vi "UHR-Fleezers Control (host) - 12.7.vi"() -> ()   [LabVIEW 2012] (continued)
  T21 = enum16{"empty", "write", "read oldest (queue)", "read newest (stack)", "read all"}
  T22 = cluster{"New Image":T2, "New Image":T2, "New Image":T2, "New Image":T2, "New Image":T2}
  T23 = typedef "XDNodeRunTimeDep.lvlib/timing_clust.ctl" = cluster{"Expected End [f-1]":u64, "Actual End [f-1]":u64, "Finished Late? [f-1]":bool, "Expected End [i-1]":u64, "Actual End [i-1]":u64, "Finished Late? [i-1]":bool, "Expected Start [i]":u64, "Actual Start [i]":u64, "Expected Start [f]":u64, "Actual Start [f]":u64, "Source Name":string, "Structure Name":string, "Period":i64, "Deadline":i64, "Offset":i64, "Start":i64, "Priority":i32, "Timeout":i32, "Mode":T24, "Wakeup Reason":T25, "Error":errorcluster, "Source Type":string, "Secondary Source Type":string, "Global End Time":u64, "Global Start Time":u64, "Frame Duration":u64, "Iteration Duration":u64, "Assigned CPU":i32, "I/O Scan Engine Mode":u32}
  T24 = typedef "XDNodeRunTimeDep.lvlib/nitl_modes.ctl" = enum32{"No Change", "Process missed periods, maintain original phase", "Discard missed periods, maintain original phase", "Process missed periods, ignore original phase", "Discard missed periods, ignore original phase"}
  T25 = typedef "XDNodeRunTimeDep.lvlib/wakeup.ctl" = enum32{"Normal", "Aborted", "Asynchronous wakeup", "Timing source error", "Timed loop error", "Timeout"}
  T26 = enum32{"Status", "Sample Stage", "Syringe Pump", "Trap Control (RF)", "APD Counting", "Fluorescence Laser Control", "Trap AI", "Video", "FPGA"}
  T27 = enum32{"Status", "Sample Stage", "Syringe Pump", "Trap Control (RF)", "APD Counting", "Fluorescence Laser Control", "Trap AI", "Video", "FPGA", "Misc. Configuration"}
  T28 = enum16{"big-endian, network order", "native, host order", "little-endian"}
  T29 = enum16{"open", "replace", "create", "open or create", "replace or create", "replace or create with confirmation"}
  T30 = cluster{"Scan Range AOD (nm) 2":dbl, "Step Size AOD (nm) 2":dbl, "Scan Speed AOD (nm/s) 2":dbl, "Number of scans (AOD) 2":u16, "Label":string}
  T31 = cluster{"[0]":dbl, "[1]":dbl, "[2]":dbl, "[3]":dbl, "[4]":dbl, "[5]":dbl}
  T32 = cluster{"Diameter (mm)":dbl, "Units":dbl, "Volume":dbl, "Rate":dbl}
  T33 = cluster{"Left":i32, "Top":i32, "Width":u32, "Height":u32}
  T34 = cluster{cluster{"Left":i32, "Top":i32, "Width":u32, "Height":u32}}[]
  T35 = enum32{"Normal Display", "Dual Display (APD)", "FFT", "High Res Display"}
  T36 = cluster{"Origin Pixel":cluster{"X":sgl, "Y":sgl}, "Angle Relative to Horizontal (deg)":sgl, "Axis Reference":u32}
  T37 = typedef "Simple Grid Descriptor" = cluster{"X Step":sgl, "Y Step":sgl, "Unit":T38}
  T38 = typedef "Image Unit" = enum32{"Undefined", "Angström", "Micrometer", "Millimeter", "Centimeter", "Meter", "Kilometer", "Microinch", "Inch", "Feet", "Nautical miles", "Standard miles", "Steps"}
  T39 = cluster{"averaging mode":u16, "weighting mode":u16, "number of averages":u32}
  T40 = cluster{"dB On (F)":bool, "unwrap phase (F)":bool, "convert to degree (F)":bool}
  T41 = cluster{string, string, string, string, string, string, string, string}
  T42 = cluster{string, string, string, string, string, string, string, string, string, string, string, string}
  T43 = cluster{string, string, string, string, string, string, string, string, string, string, string, string, string}
  T44 = cluster{string, string, string, string, string, string, string, string, string, string, string, string, string, string}
  T45 = cluster{"BD 1 Frequency 1 (MHz)":dbl, "BD 1 Frequency 2 (MHz)":dbl}
  T46 = cluster{"f0":dbl, "df":dbl, "magnitude":dbl[]}[][]
  T47 = cluster{"Comment (data description)":string, "Channel 1 Buffer":string, "Channel 2 Buffer":string, "Channel 3 Buffer":string, "Title":string, "DNA Construct":string, "Bead diameter":dbl, "Name":string}
  T48 = enum32{"setting", "request", "request control", "info", "statistics", "system settings", "I/O sub system", "HRT control", "camera descriptions", "device specific data", "event sub system settings", "event sub system results", "image memory manager"}
  T49 = typedef "AviRefnum.ctl" = refnum<k1>
  T50 = typedef "imagedata.ctl" = cluster{"image type":i32, "image depth":i32, "image":u8[], "mask":u8[], "colors":u32[], "Rectangle":cluster{"left":i16, "top":i16, "right":i16, "bottom":i16}}
diagram:
  w8 = u16 10 items=["1.0"=10, "1.5"=15, "2.0"=20] ("stop bits (10: 1 bit)")
  w75 = u16 20 items=["1.0"=10, "1.5"=15, "2.0"=20] ("stop bits (10: 1 bit)")
  w78 = u16 20 items=["1.0"=10, "1.5"=15, "2.0"=20] ("stop bits (10: 1 bit)")
  w104 = u16 20 items=["1.0"=10, "1.5"=15, "2.0"=20] ("stop bits (10: 1 bit)")
  w14 = T18 2 items=["Grayscale (U8)", "Grayscale (I16)", "Grayscale (SGL)", "Complex (CSG)", "RGB (U32)", "HSL (U32)", "RGB (U64)", "Grayscale (U16)"] ("Image Type")
  w234 = 10.0 ("y")
  w233 = 32767.0 ("y")
  w249 = 6.0  # clock mult.
  w250 = 49152000.0  # TCXO frequ.
  # "What are these?"
  # "I don't think you need to do this.\nEverytime you want to adjust phase you always set this anyway.\nSince we removed the separate +/- controls.\n\nHaven't added for added fl lasers.  Should remove this code."
  # "Bottom 1 Harvard"
  # "Top 3 Harvard"
  # "Center Harvard"
  # "Bottom 1 Harvard"
  # "Top 3 Harvard"
  # "Center Harvard"
  n1 = Build Array("DIO count 1 (ticks)", "DIO count 2 (ticks)", "DIO count 3 (ticks)") -> (w155:u16[])
  n2 = xnode "Open FPGA VI Reference"("resource name"=T19 "750kHzDAQ") -> ("FPGA VI Reference Out"=w258:T20, "error out"=w257:errorcluster)  [unwired: 1 in]
  n3 = local read "AO1"() -> (w228:dbl)
  n4 = local read "AO2"() -> (w227:dbl)
  n5 = local read "Scan Increment (MHz)"() -> (w245:dbl)
  n6 = local read "Continuous MCL Scanning"() -> (w215:bool)
  n7 = local read "Fast Scan Dir"() -> (w214:bool)
  n8 = xnode "Invoke Method"("FPGA VI Reference In"=w258, "error in"=w257) -> ("FPGA VI Reference Out"=w18:T20, "error out"=w174:errorcluster)
  n9 = local read "Number of scans (MCL)"() -> (w216:u64)
  n10 = Multiply(x=w228, y=w233) -> (x*y=w230:dbl)
  n11 = Multiply(x=w227, y=w233) -> (x*y=w232:dbl)
  n12 = Divide(x=w230, y=w234) -> (x/y=w229:dbl)
  n13 = Divide(x=w232, y=w234) -> (x/y=w231:dbl)
  n14 = To Word Integer(number=w229) -> (16bit integer=w226:i16)
  n15 = To Word Integer(number=w231) -> (16bit integer=w225:i16)
  n16 = Not(x=w214) -> (.not. x?=w209:bool)
  n17 = local read "Cycles/step (MCL)"() -> (w217:u64)
  n18 = Multiply(x=w245, y=1000.0) -> (x*y=w252:dbl)
  n19 = local read "Scan steps (MCL)"() -> (w218:u64)
  n20 = local read "Desired Scan Incr (V)"() -> (w220:dbl)
  n21 = Scale By Power Of 2(n=48, x=w252) -> (x*2^n=w253:dbl)
  n22 = Unbundle By Name(cluster{"output high":i16, "output low":i16} {"output high"=3000, "output low"=0} ("FB output range 1")) -> ("output high"=w56:i16, "output low"=w55:i16)
  n23 = Multiply(x=w250, y=w249) -> (x*y=w248:dbl)
  n24 = Divide(x=w253, y=w248) -> (x/y=w247:dbl)
  n25 = local read "Setpoints (V)"() -> (w264:cluster{"Set 1":dbl, "Set 2":dbl})
  n26 = To Quad Integer(1:w247) -> (0:w244:i64)
  n27 = Divide(x=40000000.0, y="AI Count (ticks)") -> (x/y=w205:dbl)
  n28 = Multiply(x=w220, y=32767.0) -> (x*y=w222:dbl)
  n29 = local read "Trap Intensity PID Gains"() -> (w259:T9)
  n30 = local write "Trap Pos FIFO Timeout"(u16 0 ("Trap Pos FIFO Timeout")) -> ()
  n31 = local read "Number Interlace Sets"() -> (w148:u8)
  n32 = Split 1D Array(array=w155, index=w148) -> (first subarray=w157:u16[])  [unwired: 1 out]
  n33 = Add Array Elements(numeric array=w157) -> (sum=w156:u16)
  n34 = local read "# Samples/channel"() -> (w237:u32)
  n35 = local read "Number of F/B Scans (AOD)"() -> (w238:u16)
  n36 = local read "Not-Interlacing Set"() -> (w147:enum32{"Set 1", "Set 2", "Set 3"})
  n37 = To Unsigned Byte Integer(number=w147) -> (unsigned 8bit integer=w153:u8)
  n38 = Index Array(array=w155, index=w153) -> (element=w154:u16)
  n39 = local read "Feedback On/Off"() -> (w267:cluster{"Set 1":bool, "Set 2":bool})
  n40 = local read "BD 2 Delay (Ticks)"() -> (w1:u8)
  n41 = local read "BD 1 Delay (ticks)"() -> (w2:u8)
  n42 = local read "Scan steps (AOD)"() -> (w243:u64)
  n43 = local read "All FB On/Off"() -> (w268:bool)
  n44 = local read "Cycles/step (AOD)"() -> (w242:u64)
  n45 = local write "AI rate (Hz)"(w205) -> ()
  n46 = Divide(x=w222, y=10.0) -> (x/y=w221:dbl)
  n47 = Multiply(x=w243, y=w242) -> (x*y=w241:u64)
  n48 = Unbundle By Name(w259) -> ("proportional gain (Kc)"=w60:i16, "integral gain (Kc*Ts/Ti)"=w59:i16, "derivative gain (Kc*Td/Ts)"=w58:i16)
  n49 = property on="AI Count (ticks)" class="DigNum (strict)"("Val(Sgnl)"="AI Count (ticks)") -> ()  [unwired: 2 in, 2 out]
  n50 = Multiply(x=3276.7, y=w264) -> (x*y=w263:cluster{"Set 1":dbl, "Set 2":dbl})
  n51 = To Word Integer(number=w221) -> (16bit integer=w219:i16)
  n52 = Multiply(x=w241, y=u64 2) -> (x*y=w239:u64)
  n53 = Divide(x=w205, y="FPGA Ave.") -> (x/y=w206:dbl)
  n54 = To Word Integer(number=w263) -> (16bit integer=w262:cluster{"Set 1":i16, "Set 2":i16})
  n55 = Multiply(x=w239, y=w238) -> (x*y=w236:u64)
  n56 = local read "Sets to FIFO (Traps)"() -> (w64:T15)
  n57 = local write "Ave. Rate (Hz)"(w206) -> ()
  n58 = Divide(x=w236, y=w237) -> (x/y=w235:dbl)
  n59 = Unbundle By Name(w262) -> ("Set 1"=w261:i16, "Set 2"=w260:i16)
  n60 = local read "2D or 1D Scan"() -> (w166:bool)
  n61 = local write "Data points/scans"(w236) -> ()
  n62 = local read "Scan BD"() -> (w254:bool)
  n63 = And(x=w267, y=w268) -> (x .and. y?=w266:cluster{"Set 1":bool, "Set 2":bool})
  n64 = local write "Data points/scan (f/b)"(w239) -> ()
  n65 = Reciprocal(x=w206) -> (1/x=w207:dbl)
  n66 = local read "N Acq Sets (Traps + Fl.)"() -> (w198:i16)
  n67 = local write "N sets should be saved"(w235) -> ()
  n68 = Unbundle By Name(w266) -> ("Set 1"=w270:bool, "Set 2"=w269:bool)
  n69 = local read "Interlace"() -> (w149:bool)
  n70 = Select(t=w156, s=w149, f=w154) -> (s? t:f=w146:u16)
  n71 = local write "Update Count (MCL)"(w146) -> ()
  n72 = local write "Total Counts (ticks)"(w146) -> ()
  n73 = local write "Ave. Period (s)"(w207) -> ()
  n74 = Unbundle By Name(w64) -> ("Set 1"=w63:bool, "Set 2"=w62:bool, "Set 3"=w61:bool)
  n75 = property on="2D or 1D Scan" class="Bool (strict)"("Val(Sgnl)"=w166) -> ()  [unwired: 2 in, 2 out]
  n76 = xnode "Read/Write Control"("FPGA VI Reference In"=w165, "error in"=w174, "ai count"="AI Count (ticks)", "Interlace ON/OFF"=w149, "Number Interlace Cycles"=w148, "Set 1"=w63, "Set 2"=w62, "Set 3"=w61, "FB On/Off Set 1"=w270, "FB On/Off Set 2"=w269, "Interlace Off Parameters"=w147, "FB Setpoint Set 1"=w261, "FB Setpoint Set 2"=w260, "P1"=w60, "I1"=w59, "D1"=w58, "FB1 output high"=w56, "FB1 output low"=w55, "Cycles per step"=w242, "Scan BD"=w254, "Number of scans"=w238, "Scan steps"=w243, "Scan freq.  increment"=w244, "AO1"=w226, "AO2"=w225, "Scan freq.  increment (MCL)"=w219, "Scan steps (MCL)"=w218, "Cycles per step (MCL)"=w217, "Number of scans (MCL)"=w216, "MCL count"=w146, "Cont. Scan (MCL)"=w215, "MCL Scan Axis"=w209, "1D or 2D Scan?"=w166, "N of AI1 Int Acq Sets"=w198, "Amp switch delay"="Amp switch delay", "Swap F1 and F2"="Swap F1 and F2", "APD to FIFO"=FALSE, "DIO count 1 (ticks)"="DIO count 1 (ticks)", "DIO count 2 (ticks)"="DIO count 2 (ticks)", "DIO count 3 (ticks)"="DIO count 3 (ticks)", "BD 1 Delay (ticks)"=w2, "BD 2 Delay (Ticks)"=w1) -> ("FPGA VI Reference Out"=w20:T20, "error out"=w19:errorcluster)  [unwired: 1 in]
  n77 = local read "Laser interlacing mode"() -> (w145:enum32{"Laser ON", "Laser OFF", "Interlace"})
  n78 = local read "Green Laser ON"() -> (w144:bool)
  n79 = local read "Trap Pos. FB Range"() -> (w54:T12)
  n80 = local read "Trap Pos. FB Gains"() -> (w53:T11)
  n81 = Multiply(x="Green Intensity % (FB OFF)", y=655.35) -> (x*y=w137:dbl)
  n82 = local read "Invert laser interlacing"() -> (w33:bool)
  n83 = local read "Trap Pos. AI1 X Pre-scale"() -> (w92:u16)
  n84 = Multiply(x="Green FB Setpoint (mV)", y=3.2767) -> (x*y=w134:dbl)
  n85 = local read "Trap Pos FB Int Count"() -> (w86:u16)
  n86 = local read "Differential FB?"() -> (w80:bool)
  n87 = local read "Neg. TTrig FPGA"() -> (w82:bool)
  n88 = Multiply(x="Red FB Setpoint (mV)", y=3.2767) -> (x*y=w41:dbl)
  n89 = To Unsigned Word Integer(number=w137) -> (unsigned 16bit integer=w135:u16)
  n90 = Multiply(x="Red Intensity % (FB OFF)", y=655.35) -> (x*y=w37:dbl)
  n91 = To Word Integer(number=w134) -> (16bit integer=w132:i16)
  n92 = Unbundle By Name("Green FB Gains") -> ("proportional gain (Kc)"=w45:i16, "integral gain (Kc*Ts/Ti)"=w44:i16, "derivative gain (Kc*Td/Ts)"=w43:i16)
  n93 = Unbundle By Name("Red FB Gains") -> ("proportional gain (Kc)"=w30:i16, "integral gain (Kc*Ts/Ti)"=w29:i16, "derivative gain (Kc*Td/Ts)"=w28:i16)
  n94 = case shown="False" w144 {
    tunnel: w145 -> [_ w296]
    tunnel: [enum32{"Laser ON", "Laser OFF", "Interlace"}."Laser OFF" ("Green laser mode") w296] -> w32
    frame False {
    }
    frame True {
    }
  }
  n95 = To Word Integer(number=w41) -> (16bit integer=w38:i16)
  n96 = Unbundle By Name(w53) -> ("proportional gain (Kc)"=w49:fxp<+/-,16,8>, "integral gain (Kc*Ts/Ti)"=w48:fxp<+/-,16,8>, "derivative gain (Kc*Td/Ts)"=w47:fxp<+/-,16,8>)
  n97 = To Unsigned Word Integer(number=w37) -> (unsigned 16bit integer=w34:u16)
  n98 = Unbundle By Name(w54) -> ("output high"=w52:fxp<+/-,16,1>, "output low"=w50:fxp<+/-,16,1>)
  n99 = local read "Trap Pos FB Monitor\nT1 or T2"() -> (w97:bool)
  n100 = local read "Trap Pos FB Negate Action"() -> (w96:bool)
  n101 = local read "Trap Pos. FB Offset Factor"() -> (w95:i64)
  n102 = local read "Trap Pos. FB Mult Factor"() -> (w94:i64)
  n103 = xnode "Read/Write Control"("FPGA VI Reference In"=w20, "error in"=w19, "Invert GI 2"=w33, "Operating Mode 2"=w32, "P3"=w45, "I3"=w44, "D3"=w43, "Green FB Setpoint"=w132, "Green FB On/Off"="Green FB On/Off", "Current Out"=w135, "Green int current ON count adj"="Green int current ON count adj", "Operating Mode"=w32, "Invert GI"=w33, "Trap Pos FB Monitor T1 or T2"=w97, "Trap Pos FB Negate Action"=w96, "Trap Pos. FB Offset Factor"=w95, "Trap Pos. FB Mult Factor"=w94, "Force feedback"=FALSE, "AI1 X Scale"=w92, "Trap Pos to FIFO"=TRUE, "Trap Pos FB Int Count"=w86, "TTrig Negate Pos"=w82, "FB Trig Integrate"="FB Trig Integrate", "Diff FB Measurement?"=w80, "Negate Diff?"="Negate Diff?", "P2"=w49, "I2"=w48, "D2"=w47, "FB2 output high"=w52, "FB2 output low"=w50, "Red FB Setpoint"=w38, "RI Current Out"=w34, "Red Laser Operating Mode"=w32, "RI Operating Mode 2"=w32, "Invert RI 2"=w33, "Invert RI"=w33, "P4"=w30, "I4"=w29, "D4"=w28, "Red FB On/Off"="Red FB On/Off") -> ("FPGA VI Reference Out"=w24:T20, "error out"=w26:errorcluster)
  n104 = stacked-sequence {
    tunnel: w26 -> [_ _ _ w307]
    tunnel: [_ _ _ w307] -> w25
    tunnel: w24 -> [_ _ _ w308]
    tunnel: [_ _ _ w308] -> w23
    frame #0 {
      w297 = T21."empty" ("mode")
      # "Clear external fluorescence triggering FIFO"
      # "APD loop counts"
      # "Fluorescence loop counts (rates)"
      n105 = local read "APD Integration Time (s)"() -> (w299:dbl)
      n106 = local read "Interlace ON count"() -> (w300:u16)
      n107 = call "Smart Buffer (DBL) 1.vi"("mode"=w297) -> ()  [unwired: 5 in, 6 out]
      n108 = call "Smart Buffer (DBL) 2.vi"("mode"=w297) -> ()  [unwired: 5 in, 6 out]
      n109 = property on="APD Integration Time (s)" class="DigNum (strict)"("Val(Sgnl)"=w299) -> ()  [unwired: 2 in, 2 out]
      n110 = property on="Interlace ON count" class="DigNum (strict)"("Val(Sgnl)"=w300) -> ()  [unwired: 2 in, 2 out]
      "Number of APDs" <- 3.0 ("Number of APDs")
    }
    frame #1 {
      # "Number of APDs affects\nAPD DMA transfer"
      # "General settings for all lasers:"
      # "And includes all laser\nON/OFF settings"
      # "Fluorescent lasers settings:"
      # "Blue laser settings:"
      n111 = local read "Laser interlacing mode"() -> (w302:enum32{"Laser ON", "Laser OFF", "Interlace"})
      n112 = local read "Invert laser interlacing"() -> (w301:bool)
      n113 = local read "Blue FB On/Off"() -> (w303:bool)
      n114 = property on="Blue FB On/Off" class="Bool (strict)"("Val(Sgnl)"=w303) -> ()  [unwired: 2 in, 2 out]
      n115 = property on="Invert laser interlacing" class="Bool (strict)"("Val(Sgnl)"=w301) -> ()  [unwired: 2 in, 2 out]
      n116 = property on="Laser interlacing mode" class="RadioBtnsControl (strict)"("Val(Sgnl)"=w302) -> ()  [unwired: 2 in, 2 out]
    }
    frame #2 {
      w304 = path "C:/Home/wheeler/Comstock-LabView-Link.udl" ("connection information")
      # "Initialize the database connection"
      n117 = call-poly <vilib>:"DB Tools Open Connection.vi"("connection information"=w304) -> ("connection reference"=w305:T17)  [unwired: 7 in, 1 out]
      "connection reference" <- w305
      n118 = local write "connection reference"(w305) -> ()
      n119 = local write "Database link"(w304) -> ()
    }
    frame #3 {
      n120 = Wait (ms)(milliseconds to wait=u32 1000) -> ()  [unwired: 1 out]
    }
  }
  n121 = local write "Offset (nm)"(0.0 ("Offset (nm)")) -> ()
  n122 = local write "Bead Mean (nm)"(0.0 ("Bead Mean (nm)")) -> ()
  n123 = case shown="\"2axisAOD\"" "1axis AOM vs 2 axis AOD" {
    tunnel: [T16 {"Minimum"=0.0, "Maximum"=40.0, "Increment"=1.0} ("Min Max Inc") T16 {"Minimum"=60.0, "Maximum"=90.0, "Increment"=1.0} ("Min Max Inc")] -> w5
    tunnel: [T16 {"Minimum"=0.0, "Maximum"=45.0, "Increment"=1.0} ("Data Entry Limits") T16 {"Minimum"=0.0, "Maximum"=50.0, "Increment"=1.0} ("Data Entry Limits")] -> w3
    frame "2axisAOD" {
      # "Amp Limits"
      # "Freq Limits"
    }
    frame "1axis", Default {
      # "Amp Lmits"
      # "Freq Limits"
    }
  }
  n124 = xnode "Invoke Method"("FPGA VI Reference In"=w23, "error in"=w25, "Requested Depth"="Trap AI FIFO Depth") -> ("FPGA VI Reference Out"=w100:T20, "error out"=w99:errorcluster)  [unwired: 1 out]
  n125 = xnode "Invoke Method"("FPGA VI Reference In"=w100, "error in"=w99, "Requested Depth"="Trap Position FIFO Depth") -> ("FPGA VI Reference Out"=w88:T20, "error out"=w87:errorcluster)  [unwired: 1 out]
  n126 = flat-sequence "Safety limits on RF frequencies and amplitudes (for AOM protection)" {
    tunnel: w18 -> [w317]
    tunnel: [w317] -> w165
    tunnel: [w314] -> w164
    tunnel: [w313] -> w163
    tunnel: [w315] -> w161
    tunnel: [w316] -> w162
    tunnel: w5 -> [w314]
    tunnel: w3 -> [w313]
    frame #0 {
      w316 = T16 {"Minimum"=0.0, "Maximum"=40.0, "Increment"=1.0} ("Min Max Inc")
      w315 = T16 {"Minimum"=0.0, "Maximum"=45.0, "Increment"=1.0} ("Data Entry Limits")
      n127 = property on="BD 2 Frequency 1 (MHz)" class="DigNum (strict)"("Data Range"=w316) -> ()  [unwired: 2 in, 2 out]
      n128 = property on="BD 2 Frequency 3 (MHz)" class="DigNum (strict)"("Data Range"=w316) -> ()  [unwired: 2 in, 2 out]
      n129 = property on="BD 2 Frequency 2 (MHz)" class="DigNum (strict)"("Data Range"=w316) -> ()  [unwired: 2 in, 2 out]
      n130 = property on="BD 1 Frequency 1 (MHz)" class="DigNum (strict)"("Data Range"=w314) -> ()  [unwired: 2 in, 2 out]
      n131 = property on="BD 1 Frequency 2 (MHz)" class="DigNum (strict)"("Data Range"=w314) -> ()  [unwired: 2 in, 2 out]
      n132 = property on="BD 1 Frequency 3 (MHz)" class="DigNum (strict)"("Data Range"=w314) -> ()  [unwired: 2 in, 2 out]
      n133 = property on="BD 2 Amplitude 1 (%)" class="DigNum (strict)"("Data Range"=w315) -> ()  [unwired: 2 in, 2 out]
      n134 = property on="BD 2 Amplitude 2 (%)" class="DigNum (strict)"("Data Range"=w315) -> ()  [unwired: 2 in, 2 out]
      n135 = property on="BD 2 Amplitude 3 (%)" class="DigNum (strict)"("Data Range"=w315) -> ()  [unwired: 2 in, 2 out]
      n136 = property on="BD 1 Amplitude 3 (%)" class="DigNum (strict)"("Data Range"=w313) -> ()  [unwired: 2 in, 2 out]
      n137 = property on="BD 1 Amplitude 2 (%)" class="DigNum (strict)"("Data Range"=w313) -> ()  [unwired: 2 in, 2 out]
      n138 = property on="BD 1 Amplitude 1 (%)" class="DigNum (strict)"("Data Range"=w313) -> ()  [unwired: 2 in, 2 out]
      "X RF Frequency Limits (MHz)" <- w314
      "X RF Amplitude Limits (%)" <- w313
      "Y RF Amplitude Limits (%)" <- w315
      "Y RF Frequency Limits (MHz)" <- w316
    }
  }
  n139 = xnode "Invoke Method"("FPGA VI Reference In"=w88, "error in"=w87) -> ("FPGA VI Reference Out"=w173:T20, "error out"=w172:errorcluster)  [unwired: 1 in]
  n140 = flat-sequence "Initial FPGA Loop Relative Phase Adjustment" {
    tunnel: "Initial Phase Adjustment (AI1)" -> [w332]
    tunnel: "Initial Phase Adjustment (GI)" -> [w331]
    tunnel: w173 -> [w330]
    tunnel: w172 -> [w329]
    tunnel: "Initial Phase Adj. (MCL)" -> [w328]
    tunnel: [w333] -> w182
    tunnel: [w327] -> w178
    tunnel: "Initial Phase Adjustment (APD Acq)" -> [w326]
    tunnel: "Initial Phase Adjustment (APD 1 Gate)" -> [w325]
    tunnel: "Initial Phase Adjustment (Green FB)" -> [w324]
    tunnel: "Initial Phase Adjustment (GI) 2" -> [w323]
    tunnel: "Initial Phase Adjustment (APD 2 Gate)" -> [w322]
    tunnel: "Initial Phase Adjustment (RI)" -> [w321]
    tunnel: "Initial Phase Adjustment (BI DO)" -> [w320]
    tunnel: "Initial Phase Adjustment (BI AO)" -> [w319]
    tunnel: "Initial Phase Adjustment (APD 3 Gate)" -> [w318]
    tunnel: w182 -> [w335]
    tunnel: [w336] -> w179
    tunnel: w178 -> [w336]
    tunnel: [w335] -> w177
    tunnel: w179 -> [w339]
    tunnel: w177 -> [w338]
    tunnel: [w341] -> w176
    tunnel: [w340] -> w175
    tunnel: [w343] -> w180
    tunnel: [w344] -> w181
    tunnel: w176 -> [w344]
    tunnel: w175 -> [w343]
    frame #0 {
      n141 = xnode "Read/Write Control"("FPGA VI Reference In"=w330, "error in"=w329, "Phase count adjustment"=w332, "Phase count adjustment (GI)"=w331, "Phase count adjustment (MCL)"=w328, "Phase Count Adjustment (APD Acq)"=w326, "Phase count adjustment (APD 1 Gate)"=w325, "Phase count adjustment (APD 2 Gate)"=w322, "Phase count adjustment (Green FB)"=w324, "Phase count adjustment (GI) 2"=w323, "Phase count adjustment (RI)"=w321, "Phase count adjustment (BI AO)"=w319, "Phase count adjustment (BI D)"=w320, "Phase count adjustment (APD 3 Gate)"=w318) -> ("FPGA VI Reference Out"=w327:T20, "error out"=w333:errorcluster)
    }
    frame #1 {
      n142 = Wait (ms)(milliseconds to wait=u32 100) -> ()  [unwired: 1 out]
    }
    frame #2 {
      w337 = TRUE
      n143 = xnode "Read/Write Control"("FPGA VI Reference In"=w339, "error in"=w338, "+ phase"=w337, "+ phase (GI)"=w337, "+ phase (MCL)"=w337, "+ phase (APD Acq)"=w337, "+ phase (APD 1 Gate)"=w337, "+ phase (APD 2 Gate)"=w337, "+ phase (Green FB)"=w337, "+ phase (GI) 2"=w337, "+ phase (RI)"=w337, "+ phase (BI AO)"=w337, "+ phase (BI D)"=w337, "+ phase (APD 3 Gate)"=w337) -> ("FPGA VI Reference Out"=w340:T20, "error out"=w341:errorcluster)
    }
    frame #3 {
      n144 = Wait (ms)(milliseconds to wait=u32 100) -> ()  [unwired: 1 out]
    }
  }
  n145 = local read "Phase adj. (Green FB)"() -> (w158:i16)
  n146 = local read "Phase adj. (GI) 2"() -> (w138:i16)
  n147 = local read "Phase adjust (MCL)"() -> (w210:i16)
  n148 = local read "Phase adj. (AI1)"() -> (w212:i16)
  n149 = local read "Phase adj. (GI)"() -> (w211:i16)
  n150 = xnode "Read/Write Control"("FPGA VI Reference In"=w180, "error in"=w181, "Phase count adjustment"=w212, "Phase count adjustment (GI)"=w211, "Phase count adjustment (MCL)"=w210, "Phase Count Adjustment (APD Acq)"="Phase Adj. (APD Acq)", "Phase count adjustment (APD 1 Gate)"="Phase Adj. (APD 1 Gate)", "Phase count adjustment (APD 2 Gate)"="Phase Adj. (APD 2 Gate)", "Phase count adjustment (Green FB)"=w158, "Phase count adjustment (GI) 2"=w138) -> ("FPGA VI Reference Out"=w124:T20, "error out"=w187:errorcluster)
  n151 = call "Initialize RF boards - interlace 3.vi"("error in"=w187, "FPGA VI Reference In"=w124) -> ("error out"=w185:errorcluster, "FPGA VI Reference Out"=w186:T20)
  n152 = call "set RF board frequency - interlace.vi"("Board 2 Frequency Limits"=w162, "Board 1 Frequency Limits"=w164, "error in"=w185, "FPGA VI Reference In"=w186, "Board 2 Frequency 3 (MHz)"="BD 2 Frequency 3 (MHz)", "Board 1 Frequency 3 (MHz)"="BD 1 Frequency 3 (MHz)", "Board 2 Frequency 2 (MHz)"="BD 2 Frequency 2 (MHz)", "Board 2 Frequency 1 (MHz)"="BD 2 Frequency 1 (MHz)", "Board 1 Frequency 2 (MHz)"="BD 1 Frequency 2 (MHz)", "Board 1 Frequency 1  (MHz)"="BD 1 Frequency 1 (MHz)") -> ("error out"=w285:errorcluster, "FPGA VI Reference Out"=w286:T20)
  n153 = call "set RF board amplitude - interlace.vi"("Board 2 Amplitude Limits"=w161, "Board 1 Amplitude Limits"=w163, "error in"=w285, "FPGA VI Reference In"=w286, "Board 2 Amplitude 3 (%)"="BD 2 Amplitude 3 (%)", "Board 1 Amplitude 3 (%)"="BD 1 Amplitude 3 (%)", "Board 2 Amplitude 2 (%)"="BD 2 Amplitude 2 (%)", "Board 2 Amplitude 1 (%)"="BD 2 Amplitude 1 (%)", "Board 1 Amplitude 2 (%)"="BD 1 Amplitude 2 (%)", "Board 1 Amplitude 1 (%)"="BD 1 Amplitude 1 (%)") -> ("error out"=w273:errorcluster, "FPGA VI Reference Out"=w274:T20)
  n154 = flat-sequence {
    tunnel: w274 -> [w354]
    tunnel: w273 -> [w353]
    tunnel: [w352] -> w278
    tunnel: [w351] -> w277
    tunnel: [w358] -> w276
    tunnel: w278 -> [w358]
    tunnel: [w357] -> w275
    tunnel: w277 -> [w357]
    tunnel: w276 -> [w367]
    tunnel: w275 -> [w366]
    tunnel: [w365] -> w17
    tunnel: [w364] -> w89
    frame #0 {
      w345 = FALSE ("Retract Pump 3")
      n155 = local read "Trap 1 (ON/OFF)"() -> (w346:bool)
      n156 = xnode "Read/Write Control"("FPGA VI Reference In"=w354, "error in"=w353, "Direct RF Box  Communication"=FALSE) -> ("FPGA VI Reference Out"=w352:T20, "error out"=w351:errorcluster)
      n157 = local write "Saving..."(FALSE ("Saving Data")) -> ()
      n158 = local write "Stop All"(FALSE ("Stop All")) -> ()
      n159 = local write "Retract Pump 1"(w345) -> ()
      n160 = local write "Retract Pump 3"(w345) -> ()
      n161 = local write "Index"(1.0 ("Index")) -> ()
      n162 = property on="Trap 1 ON" class="Bool (strict)"("Value"=w346) -> ()  [unwired: 2 in, 2 out]
      "Manipulating Trap" <- FALSE ("Manipulating Trap")
    }
    frame #1 {
      n163 = local read "Trap 2 (ON/OFF)"() -> (w356:bool)
      n164 = Wait (ms)(milliseconds to wait=u32 10) -> ()  [unwired: 1 out]
      n165 = property on="Trap 2 ON" class="Bool (strict)"("Val(Sgnl)"=w356) -> ()  [unwired: 2 in, 2 out]
    }
    frame #2 {
      n166 = local read "Scan Range (nm)"() -> (w360:dbl)
      n167 = xnode "Read/Write Control"("FPGA VI Reference In"=w367, "error in"=w366, "FPGA Controls  RF Box"=TRUE ("Direct RF Box  Communication")) -> ("FPGA VI Reference Out"=w365:T20, "error out"=w364:errorcluster)
      n168 = call "Update messages.vi"("Message to add"="UHR-Fleezers ready.", "Old message string"="") -> ("New message string"=w363:string)
      n169 = local write "Messages"(w363) -> ()
      n170 = property on="Scan Range (nm)" class="DigNum (strict)"("Val(Sgnl)"=w360) -> ()  [unwired: 2 in, 2 out]
    }
  }
  n171 = Subtract(x="BD 1 Frequency 1 (MHz)", y="BD 1 Frequency 2 (MHz)") -> (x-y=w197:dbl)
  n172 = Subtract(x="BD 2 Frequency 1 (MHz)", y="BD 2 Frequency 2 (MHz)") -> (x-y=w196:dbl)
  n173 = Square(x=w196) -> (x^2=w194:dbl)
  n174 = Square(x=w197) -> (x^2=w195:dbl)
  n175 = Add(x=w195, y=w194) -> (x+y=w193:dbl)
  n176 = Square Root(x=w193) -> (sqrt(x)=w192:dbl)
  n177 = local write "Trap Delta (MHz)"(w192) -> ()
  n178 = call-poly "VISA Configure Serial Port"("VISA resource name"="VISA resource name", "baud rate (9600)"=u32 115200, "stop bits (10: 1 bit)"=w8) -> ("VISA resource name out"=w7:refnum<visa-resource-name>, "error out"=w6:errorcluster)  [unwired: 4 in, 7 out]
  n179 = call-poly "VISA Configure Serial Port"("VISA resource name"="Bottom  1 Harvard Syringe Pump Serial Port", "baud rate (9600)"=u32 115200, "stop bits (10: 1 bit)"=w75) -> ("VISA resource name out"=w71:refnum<visa-resource-name>, "error out"=w70:errorcluster)  [unwired: 4 in, 7 out]
  n180 = call-poly "VISA Configure Serial Port"("VISA resource name"="Top 3 Harvard Syringe Pump Serial Port", "baud rate (9600)"=u32 115200, "stop bits (10: 1 bit)"=w78) -> ("VISA resource name out"=w73:refnum<visa-resource-name>, "error out"=w72:errorcluster)  [unwired: 4 in, 7 out]
  n181 = call-poly "VISA Configure Serial Port"("VISA resource name"="Sample Chamber Stage Serial Port") -> ("VISA resource name out"=w119:refnum<visa-resource-name>, "error out"=w120:errorcluster)  [unwired: 5 in, 8 out]
  "Stage Control Serial Error" <- w120
  n182 = local write "Blue Error Out"(w6) -> ()
  n183 = call-poly "VISA Configure Serial Port"("VISA resource name"="Center Harvard Syringe Pump Serial Port", "baud rate (9600)"=u32 115200, "stop bits (10: 1 bit)"=w104) -> ("VISA resource name out"=w101:refnum<visa-resource-name>, "error out"=w102:errorcluster)  [unwired: 4 in, 7 out]
  n184 = call "IMAQ Create"("Image Name"="APD 1 Image", "Image Type"=w14) -> ("New Image"=w110:T2)  [unwired: 3 in, 1 out]
  n185 = call "IMAQ Create"("Image Name"="APD 2 Image", "Image Type"=w14) -> ("New Image"=w109:T2)  [unwired: 3 in, 1 out]
  n186 = call "IMAQ Create"("Image Name"="APD 3 Image", "Image Type"=w14) -> ("New Image"=w13:T2)  [unwired: 3 in, 1 out]
  n187 = call "IMAQ Create"("Image Name"="Det. X Image", "Image Type"=w14) -> ("New Image"=w108:T2)  [unwired: 3 in, 1 out]
  n188 = call "IMAQ Create"("Image Name"="Det. Y Image", "Image Type"=w14) -> ("New Image"=w107:T2)  [unwired: 3 in, 1 out]
  n189 = Bundle("New Image"=w110, "New Image"=w109, "New Image"=w13, "New Image"=w108, "New Image"=w107) -> (w106:T22)  [unwired: 1 in]
  n190 = node-c288() -> (w115:T23)  [unwired: 4 in]
  n191 = node-c288(3 ("Processor")) -> (w126:T23)  [unwired: 3 out]
  n192 = node-c288(2 ("Processor")) -> (w128:T23)  [unwired: 3 out]
  n193 = node-c288() -> (w130:T23)  [unwired: 4 out]
  n194 = node-c288(i64 1 ("Period"), 1 ("Processor")) -> (w201:T23)  [unwired: 2 out]
  n195 = timed-loop "Run Scripts, including: stage motion" {
    tunnel: w120 -> [w376]
    tunnel: w119 -> [w377]
    tunnel: [w377] -> w118
    tunnel: [w376] -> w117
    timing: w115 -> [_]
    timing-out: [_] -> w114
    tunnel: w101 -> [w375]
    tunnel: w102 -> [w374]
    tunnel: w73 -> [w371]
    tunnel: w72 -> [w370]
    tunnel: w71 -> [w372]
    tunnel: w70 -> [w373]
    tunnel: w7 -> [w369]
    stop <- w378 stop-if-true
    n196 = node-c288() -> ()  [unwired: 1 in, 1 out]
    n197 = event shown="[5] \"Blue Laser Modluation Mode\": Value Change" {
      selector: _ -> [_ _ _ _ _ _ _ _ _ _ _ _ _ _ _ _ _ _ _ _ _ _ _]
      dyn-events: _ -> [_ _ _ _ _ _ _ _ _ _ _ _ _ _ _ _ _ _ _ _ _ _ _]
      timeout: _ -> [_ _ _ _ _ _ _ _ _ _ _ _ _ _ _ _ _ _ _ _ _ _ _]
      tunnel: ["Set Position" "Move to Position" _ _ _ _ _ _ "Read Harvard" _ _ _ _ _ _ "Got ADig bead" "Force FB Data\nScript" _ "Got DNA bead" "Take Stepping Data" _ "Take Detection Laser\nImage" _] -> _
      tunnel: [_ _ _ _ _ _ _ _ _ _ _ _ _ _ _ _ _ _ _ _ _ _ w1072] -> w378
      tunnel: w376 -> [w396 w404 w417 w447 _ _ _ _ _ w563 w603 w684 w713 w845 w871 _ w907 _ _ _ _ _ _]
      tunnel: w377 -> [w397 w405 w418 w448 _ _ _ _ _ w564 w604 w685 w714 w846 w872 _ w908 _ _ _ _ _ _]
      tunnel: w375 -> [_ _ _ _ _ _ _ _ w548 _ _ _ _ _ _ _ _ _ _ _ _ _ _]
      tunnel: w374 -> [_ _ _ _ _ _ _ _ w547 _ _ _ _ _ _ _ _ _ _ _ _ _ _]
      tunnel: w373 -> [_ _ _ _ _ _ _ _ _ _ _ _ _ _ _ _ _ _ _ _ _ _ _]
      tunnel: w372 -> [_ _ _ _ _ _ _ _ _ _ _ _ _ _ _ _ _ _ _ _ _ _ _]
      tunnel: w371 -> [_ _ _ _ _ _ _ _ _ _ _ _ _ _ _ _ _ _ _ _ _ _ _]
      tunnel: w370 -> [_ _ _ _ _ _ _ _ _ _ _ _ _ _ _ _ _ _ _ _ _ _ _]
      tunnel: w369 -> [_ _ _ _ w475 w503 w527 w538 _ _ _ _ _ _ _ _ _ _ _ _ _ _ w1071]
      event "Set Position", "Set Position 2", "Set Position 3", "Set Position 4", "Set Position 5", "Set Position 1": Value Change {
        n198 = event-data() -> ()  [unwired: 1 in, 5 out]
        n199 = Build Array("Set Position 1", "Set Position 2", "Set Position 3", "Set Position 4", "Set Position 5") -> (w395:bool[])
        n200 = Boolean Array To Number(Boolean array=w395) -> (number=w394:u32)
        n201 = Logarithm Base 2(1:w394) -> (0:w386:dbl)
        n202 = call "Read Stage Position.vi"("error in"=w396, "VISA resource name in"=w397) -> ("Current Position"=w401:cluster{dbl, dbl, dbl}, "error out"=w400:errorcluster)  [unwired: 2 out]
        n203 = Decrement(x="Position") -> (x-1=w384:dbl)
        n204 = Greater Or Equal?(x=w386, y=0.0) -> (x >= y?=w387:bool)
        n205 = Cluster To Array(cluster=w401) -> (array=w398:dbl[])
        n206 = local write "Stage Control Serial Error"(w400) -> ()
        n207 = Select(t=w386, s=w387, f=w384) -> (s? t:f=w383:dbl)
        n208 = Increment(x=w383) -> (x+1=w382:dbl)
        n209 = Build Array (concatenate)(w382, w398) -> (w381:dbl[])
        n210 = Replace Array Subset(array="Saved Stage Positions", new element=w381, index (row)=w383) -> (w399:dbl[][])  [unwired: 1 in]
        n211 = local write "Saved Stage Positions"(w399) -> ()
      }
      event "Move to Position": Value Change {
        n212 = event-data() -> ()  [unwired: 1 in, 5 out]
        n213 = flat-sequence {
          tunnel: w405 -> [w409]
          tunnel: w404 -> [w408]
          frame #0 {
            n214 = local read "Saved Stage Positions"() -> (w411:dbl[][])
            n215 = local read "Position"() -> (w410:dbl)
            n216 = local write "Stage Moving"(TRUE ("Stage Moving")) -> ()
            n217 = call "move to saved stage position.vi"("error in"=w408, "Stage VISA resource name in"=w409, "Position"=w410, "Saved Stage Positions"=w411) -> ("error out"=w407:errorcluster)  [unwired: 1 out]
            n218 = local write "Stage Control Serial Error"(w407) -> ()
          }
          frame #1 {
            n219 = call <vilib>:"Beep.vi"() -> ()  [unwired: 3 in, 9 out]
            n220 = local write "Stage Moving"(FALSE ("Stage Moving")) -> ()
          }
        }
      }
      event "Move Cap. 1 (DNA Bottom)": Value Change {
        n221 = event-data() -> ()  [unwired: 1 in, 5 out]
        n222 = local write "Move Cap. 1 (DNA Bottom)"(FALSE ("Move Cap. 1 (DNA Right)")) -> ()
        n223 = flat-sequence {
          tunnel: w417 -> [w420]
          tunnel: w418 -> [w421]
          tunnel: [w421] -> w415
          tunnel: [w420] -> w414
          tunnel: w415 -> [w423]
          tunnel: w414 -> [w422]
          frame #0 {
            n224 = property on="Sample Channel\nFlow" class="Bool (strict)"("Val(Sgnl)"="Cap 1 Samp Flow ON") -> ()  [unwired: 2 in, 2 out]
          }
          frame #1 {
            n225 = local read "Saved Stage Positions"() -> (w433:dbl[][])
            n226 = local write "Stage Moving"(TRUE ("Stage Moving")) -> ()
            n227 = Array Subset(array=w433, index (row)=0 ("index"), length (row)=1 ("length"), index (col)=1 ("index"), length (col)=3 ("length")) -> (w430:dbl[][])
            n228 = Reshape Array(w430, 3 ("dimension size")) -> (w428:dbl[])
            n229 = Array To Cluster(array=w428) -> (cluster=w427:cluster{"[0]":dbl, "[1]":dbl, "[2]":dbl})
            n230 = call "Set Stage Position.vi"("Position"=w427, "error in"=w422, "VISA resource name in"=w423) -> ("error out"=w426:errorcluster)  [unwired: 2 out]
            n231 = local write "Stage Control Serial Error"(w426) -> ()
          }
          frame #2 {
            n232 = local write "Stage Moving"(FALSE ("Stage Moving")) -> ()
            n233 = case shown="True" "Cap 1 Flow ON" {
              frame False {
              }
              frame True {
                n234 = property on="Inject Pump 1" class="Bool (strict)"("Val(Sgnl)"=TRUE ("Value (Signaling)")) -> ()  [unwired: 2 in, 2 out]
              }
            }
            n235 = call <vilib>:"Beep.vi"() -> ()  [unwired: 3 in, 9 out]
          }
          frame #3 {
            n236 = property on="Sample Channel\nFlow" class="Bool (strict)"("Val(Sgnl)"=FALSE ("Value (Signaling)")) -> ()  [unwired: 2 in, 2 out]
            n237 = local read "Cap. 2 BD T1?\n(ADig T1, DNA T2)"() -> (w440:bool)
            n238 = case shown="True" w440 {
              tunnel: "Cap 1 T ON" -> [w442 w443]
              frame False {
                n239 = property on="Trap 1 (ON/OFF)" class="Bool (strict)"("Val(Sgnl)"=w442) -> ()  [unwired: 2 in, 2 out]
              }
              frame True {
                n240 = property on="Trap 2 (ON/OFF)" class="Bool (strict)"("Val(Sgnl)"=w443) -> ()  [unwired: 2 in, 2 out]
              }
            }
            n241 = property on="Got DNA bead" class="Bool"("Key Focus"=TRUE) -> ()  [unwired: 2 in, 2 out]
          }
        }
      }
      event "Move Cap. 2 (ADig Top)": Value Change {
        n242 = event-data() -> ()  [unwired: 1 in, 5 out]
        n243 = local write "Move Cap. 2 (ADig Top)"(FALSE ("Move Cap. 2 (ADig Left)")) -> ()
        n244 = flat-sequence {
          tunnel: w447 -> [w450]
          tunnel: w448 -> [w451]
          tunnel: [w451] -> w445
          tunnel: [w450] -> w444
          tunnel: w445 -> [w454]
          tunnel: w444 -> [w453]
          frame #0 {
            n245 = property on="Sample Channel\nFlow" class="Bool (strict)"("Val(Sgnl)"="Cap 2 Samp Flow ON") -> ()  [unwired: 2 in, 2 out]
          }
          frame #1 {
            w452 = FALSE ("Value (Signaling)")
            n246 = local read "Saved Stage Positions"() -> (w464:dbl[][])
            n247 = local write "Stage Moving"(TRUE ("Stage Moving")) -> ()
            n248 = Array Subset(array=w464, index (row)=1 ("index"), length (row)=1 ("length"), index (col)=1 ("index"), length (col)=3 ("length")) -> (w461:dbl[][])
            n249 = Reshape Array(w461, 3 ("dimension size")) -> (w459:dbl[])
            n250 = property on="Trap 1 (ON/OFF)" class="Bool (strict)"("Val(Sgnl)"=w452) -> ()  [unwired: 2 in, 2 out]
            n251 = property on="Trap 1 (ON/OFF)" class="Bool (strict)"("Val(Sgnl)"=w452) -> ()  [unwired: 2 in, 2 out]
            n252 = Array To Cluster(array=w459) -> (cluster=w458:cluster{"[0]":dbl, "[1]":dbl, "[2]":dbl})
            n253 = call "Set Stage Position.vi"("Position"=w458, "error in"=w453, "VISA resource name in"=w454) -> ("error out"=w457:errorcluster)  [unwired: 2 out]
            n254 = local write "Stage Control Serial Error"(w457) -> ()
          }
          frame #2 {
            n255 = local write "Stage Moving"(FALSE ("Stage Moving")) -> ()
            n256 = call <vilib>:"Beep.vi"() -> ()  [unwired: 3 in, 9 out]
            n257 = case shown="True" "Cap 2 Flow ON" {
              frame False {
              }
              frame True {
                n258 = property on="Inject Pump 3" class="Bool (strict)"("Val(Sgnl)"=TRUE ("Value (Signaling)")) -> ()  [unwired: 2 in, 2 out]
              }
            }
          }
          frame #3 {
            n259 = property on="Sample Channel\nFlow" class="Bool (strict)"("Val(Sgnl)"=FALSE ("Value (Signaling)")) -> ()  [unwired: 2 in, 2 out]
            n260 = case shown="False" "Cap. 2 BD T1?\n(ADig T1, DNA T2)" {
              tunnel: "Cap 2 T ON" -> [w473 w474]
              frame False {
                n261 = property on="Trap 2 (ON/OFF)" class="Bool (strict)"("Val(Sgnl)"=w473) -> ()  [unwired: 2 in, 2 out]
              }
              frame True {
                n262 = property on="Trap 1 (ON/OFF)" class="Bool (strict)"("Val(Sgnl)"=w474) -> ()  [unwired: 2 in, 2 out]
              }
            }
            n263 = property on="Got ADig bead" class="Bool"("Key Focus"=TRUE) -> ()  [unwired: 2 in, 2 out]
          }
        }
      }
      event "Initialize Blue Laser": Value Change {
        n264 = event-data() -> ()  [unwired: 1 in, 5 out]
        n265 = flat-sequence {
          tunnel: w475 -> [w494]
          frame #0 {
            n266 = Concatenate Strings("slmp ", "Blue Laser\nModulation\nPower (mW)") -> (w493:string)
            n267 = call "serial write macro.vi"("String"=w493, "Delay (ms)"="Delay (ms)", "VISA resource name"=w494) -> ("read buffer"=w482:string, "error out"=w483:errorcluster, "VISA resource name out"=w490:refnum<visa-resource-name>)
            n268 = local write "read blue buffer"(w482) -> ()
            n269 = local write "Blue Error Out"(w483) -> ()
            n270 = call "serial write macro.vi"("String"="sdmes 1", "Delay (ms)"="Delay (ms)", "VISA resource name"=w490) -> ("read buffer"=w480:string, "error out"=w481:errorcluster, "VISA resource name out"=w488:refnum<visa-resource-name>)
            n271 = local write "Blue Error Out"(w481) -> ()
            n272 = local write "read blue buffer"(w480) -> ()
            n273 = call "serial write macro.vi"("String"="sames 1", "Delay (ms)"="Delay (ms)", "VISA resource name"=w488) -> ("read buffer"=w477:string, "error out"=w479:errorcluster, "VISA resource name out"=w485:refnum<visa-resource-name>)
            n274 = local write "read blue buffer"(w477) -> ()
            n275 = local write "Blue Error Out"(w479) -> ()
            n276 = call "serial write macro.vi"("String"="l1", "Delay (ms)"="Delay (ms)", "VISA resource name"=w485) -> ("read buffer"=w476:string, "error out"=w478:errorcluster)  [unwired: 1 out]
            n277 = local write "read blue buffer"(w476) -> ()
            n278 = local write "Blue Error Out"(w478) -> ()
          }
          frame #1 {
            n279 = local write "Initialize Blue Laser"(FALSE ("Initialize")) -> ()
          }
        }
      }
      event "Blue Laser Modluation Mode": Value Change {
        # "Changes the type of modulation for the blue laser"
        n280 = event-data() -> ()  [unwired: 1 in, 5 out]
        n281 = case shown="\"Constant Power\"" "Blue Laser Modluation Mode" {
          tunnel: ["sdmes 1" w512 "sdmes 1" "sdmes 0"] -> w497
          tunnel: ["sames 1" "cp" "sames 0" "sames 1"] -> w496
          frame "Digital + Analog", Default {
          }
          frame "Constant Power" {
            n282 = local read "Blue Laser\nModulation\nPower (mW)"() -> (w515:string)
            n283 = Decimal String To Number(string=w515) -> (number=w511:i32)  [unwired: 2 in, 1 out]
            n284 = Divide(x=w511, y=1000) -> (x/y=w509:dbl)
            n285 = Number To Fractional String(number=w509) -> (F-format string=w510:string)  [unwired: 3 in]
            n286 = Concatenate Strings("p ", w510) -> (w512:string)
          }
          frame "Digital Only" {
          }
          frame "Analog Only" {
          }
        }
        n287 = local read "Delay (ms)"() -> (w506:i32)
        n288 = call "serial write macro.vi"("String"=w497, "Delay (ms)"=w506, "VISA resource name"=w503) -> ("read buffer"=w504:string, "error out"=w505:errorcluster, "VISA resource name out"=w498:refnum<visa-resource-name>)
        n289 = local write "read blue buffer"(w504) -> ()
        n290 = local write "Blue Error Out"(w505) -> ()
        n291 = local read "Delay (ms)"() -> (w501:i32)
        n292 = call "serial write macro.vi"("String"=w496, "Delay (ms)"=w501, "VISA resource name"=w498) -> ("read buffer"=w499:string, "error out"=w500:errorcluster)  [unwired: 1 out]
        n293 = local write "Blue Error Out"(w500) -> ()
        n294 = local write "read blue buffer"(w499) -> ()
      }
      event "Blue Laser\nModulation\nPower (mW)": Value Change {
        n295 = event-data() -> ()  [unwired: 1 in, 5 out]
        n296 = local read "Blue Laser\nModulation\nPower (mW)"() -> (w522:string)
        n297 = local read "Blue Laser Modluation Mode"() -> (w523:string)
        n298 = case shown="\"Constant Power\"" w523 {
          tunnel: w522 -> [w529 w536]
          tunnel: [w528 w535] -> w521
          frame "Constant Power" {
            # "Different command to change constant power instead of modulation power"
            n299 = Decimal String To Number(string=w529) -> (offset past number=w534:i32)  [unwired: 2 in, 1 out]
            n300 = Divide(x=w534, y=1000) -> (x/y=w532:dbl)
            n301 = Number To Fractional String(number=w532) -> (F-format string=w530:string)  [unwired: 3 in]
            n302 = Concatenate Strings("p ", w530) -> (w528:string)
          }
          frame Default {
            n303 = Concatenate Strings("slmp ", w536) -> (w535:string)
          }
        }
        n304 = local read "Delay (ms)"() -> (w526:i32)
        n305 = call "serial write macro.vi"("String"=w521, "Delay (ms)"=w526, "VISA resource name"=w527) -> ("read buffer"=w525:string, "error out"=w524:errorcluster)  [unwired: 1 out]
        n306 = local write "Blue Error Out"(w524) -> ()
        n307 = local write "read blue buffer"(w525) -> ()
      }
      event "Send string\nto Blue Laser": Value Change {
        n308 = event-data() -> ()  [unwired: 1 in, 5 out]
        n309 = flat-sequence {
          tunnel: w538 -> [w543]
          frame #0 {
            n310 = local read "Delay (ms)"() -> (w540:i32)
            n311 = call "serial write macro.vi"("String"="command string", "Delay (ms)"=w540, "VISA resource name"=w543) -> ("read buffer"=w541:string, "error out"=→"Blue Error Out":errorcluster)  [unwired: 1 out]
            "read blue buffer" <- w541
            n312 = String Length(string=w541) -> (length=→"length":i32)
            "command string sent" <- "command string"
          }
          frame #1 {
            n313 = local write "Send string\nto Blue Laser"(FALSE ("Send string")) -> ()
          }
        }
      }
      event "Read Harvard": Value Change {
        n314 = event-data() -> ()  [unwired: 1 in, 5 out]
        n315 = Concatenate Strings("write buffer", "\r") -> (w550:string)
        n316 = VISA Write(VISA resource name=w548, write buffer=w550, error in (no error)=w547) -> (VISA resource name out=w559:refnum<visa-resource-name>, error out=w558:errorcluster)  [unwired: 1 out]
        n317 = stacked-sequence {
          tunnel: [w562] -> w557
          tunnel: w559 -> [w562]
          tunnel: w558 -> [w561]
          tunnel: [w561] -> w552
          frame #0 {
            n318 = Wait (ms)(milliseconds to wait=50) -> ()  [unwired: 1 out]
          }
        }
        n319 = property class="Instr"(reference=w557, error in=w552) -> (reference out=w556:refnum<visa-resource-name>, error out=w554:errorcluster, "Serial Settings:Number of Bytes at Serial Port"=w555:u32)
        "Serial Settings:Number of Bytes at Serial Port" <- w555
        n320 = VISA Read(VISA resource name=w556, byte count=w555, error in (no error)=w554) -> (read buffer=w553:string)  [unwired: 3 out]
        "read buffer" <- w553
        n321 = Fract/Exp String To Number(string=w553) -> ()  [unwired: 5 out]
      }
      event "+z", "-z": Value Change {
        n322 = event-data() -> ()  [unwired: 1 in, 5 out]
        n323 = flat-sequence {
          tunnel: w563 -> [w585]
          tunnel: w564 -> [w565]
          frame #0 {
            n324 = call "Read Stage Position.vi"("error in"=w585, "VISA resource name in"=w565) -> ("Current Position"=w570:cluster{dbl, dbl, dbl}, "error out"=w583:errorcluster, "VISA resource name out"=w584:refnum<visa-resource-name>)  [unwired: 1 out]
            n325 = local read "Saved Stage Positions"() -> (w594:dbl[][])
            n326 = Divide(x="z nudge increment (um)", y=1000.0) -> (x/y=w582:dbl)
            n327 = Boolean To (0,1)(Boolean="+z") -> (0, 1=w574:i16)
            n328 = Boolean To (0,1)(Boolean="-z") -> (0, 1=w575:i16)
            n329 = Array Subset(array=w594, index (row)=1 ("index"), length (row)=1 ("length"), index (col)=1 ("index"), length (col)=3 ("length")) -> (w591:dbl[][])
            n330 = Multiply(x=w574, y=w582) -> (x*y=w578:dbl)
            n331 = Multiply(x=w575, y=w582) -> (x*y=w576:dbl)
            n332 = Unbundle(w570) -> (w568:dbl, w567:dbl, w571:dbl)
            n333 = Negate(x=w576) -> (-x=w577:dbl)
            n334 = Reshape Array(w591, 3 ("dimension size")) -> (w589:dbl[])
            n335 = Add(x=w578, y=w577) -> (x+y=w579:dbl)
            n336 = Array To Cluster(array=w589) -> ()  [unwired: 1 out]
            n337 = Add(x=w579, y=w571) -> (x+y=w569:dbl)
            n338 = Bundle(cluster=w570, w568, w567, w569) -> (w566:cluster{dbl, dbl, dbl})
            n339 = call "Set Stage Position.vi"("Position"=w566, "error in"=w583, "VISA resource name in"=w584) -> ("error out"=w588:errorcluster)  [unwired: 2 out]
            n340 = local write "Stage Moving"(TRUE ("Stage Moving")) -> ()
            n341 = local write "Stage Control Serial Error"(w588) -> ()
          }
          frame #1 {
            n342 = local write "Stage Moving"(FALSE ("Stage Moving")) -> ()
            n343 = call <vilib>:"Beep.vi"() -> ()  [unwired: 3 in, 9 out]
          }
        }
      }
      event "Cal/Data Acq. Spot": Value Change {
        n344 = event-data() -> ()  [unwired: 1 in, 5 out]
        n345 = flat-sequence {
          tunnel: w603 -> [w607]
          tunnel: w604 -> [w608]
          tunnel: [w608] -> w600
          tunnel: [w607] -> w599
          tunnel: w600 -> [w613]
          tunnel: w599 -> [w612]
          tunnel: ["Cal @ (MHz)"] -> w597
          tunnel: [w617] -> w601
          tunnel: w597 -> [w617]
          tunnel: w601 -> [w626]
          tunnel: ["W/ Offset 1"] -> w598
          tunnel: w601 -> [w647]
          tunnel: w598 -> [w645]
          frame #0 {
            n346 = property on="Sample Channel\nFlow" class="Bool (strict)"("Val(Sgnl)"="Daq spot flow on") -> ()  [unwired: 2 in, 2 out]
            n347 = Wait (ms)(milliseconds to wait=u32 250) -> ()  [unwired: 1 out]
          }
          frame #1 {
            n348 = local read "Saved Stage Positions"() -> (w610:dbl[][])
            n349 = property on="Trap Delta (MHz)" class="DigNum (strict)"("Val(Sgnl)"="Cal @ (MHz)") -> ()  [unwired: 2 in, 2 out]
            n350 = local write "Stage Moving"(TRUE ("Stage Moving")) -> ()
            n351 = call "move to saved stage position.vi"("error in"=w612, "Stage VISA resource name in"=w613, "Position"="Cal Stage Position", "Saved Stage Positions"=w610) -> ("error out"=w611:errorcluster)  [unwired: 1 out]
            n352 = local write "Stage Control Serial Error"(w611) -> ()
          }
          frame #2 {
            n353 = local write "Stage Moving"(FALSE ("Stage Moving")) -> ()
            n354 = property on="Sample Channel\nFlow" class="Bool (strict)"("Val(Sgnl)"="Flow ON during cal?") -> ()  [unwired: 2 in, 2 out]
            n355 = call <vilib>:"Beep.vi"() -> ()  [unwired: 3 in, 9 out]
          }
          frame #3 {
            n356 = Wait (ms)(milliseconds to wait=u32 1000) -> ()  [unwired: 1 out]
          }
          frame #4 {
            n357 = property on="Save Calibration" class="Bool (strict)"("Val(Sgnl)"=TRUE ("Value (Signaling)")) -> ()  [unwired: 2 in, 2 out]
          }
          frame #5 {
            n358 = Wait (ms)(milliseconds to wait=u32 2000) -> ()  [unwired: 1 out]
          }
          frame #6 {
            # "Check to see if \nsaving done"
            n359 = while {
              stop <- w622 stop-if-true
              n360 = local read "Saving..."() -> (w623:bool)
              n361 = Wait (ms)(milliseconds to wait=u32 100) -> ()  [unwired: 1 out]
              n362 = Not(x=w623) -> (.not. x?=w622:bool)
            }
          }
          frame #7 {
            n363 = case shown="True" "W/ Offset 1" {
              tunnel: w626 -> [_ w627]
              frame False {
              }
              frame True {
                n364 = stacked-sequence {
                  tunnel: w627 -> [_ _ _ _ _ _ _ w644]
                  frame #0 {
                    n365 = property on="Trap Delta (MHz)" class="DigNum (strict)"("Val(Sgnl)"="Offset 1 Start (MHz)") -> ()  [unwired: 2 in, 2 out]
                    n366 = Replace Array Subset(array=u32[] [0] ("Index Values"), new element="Offset 1 Set", index=0) -> (w628:u32[])
                    n367 = property on="Saved AOD Raster Scan Parameter Sets" class="Arr (strict)"("Index Values"=w628) -> ()  [unwired: 2 in, 2 out]
                  }
                  frame #1 {
                    n368 = Wait (ms)(milliseconds to wait=u32 200) -> ()  [unwired: 1 out]
                  }
                  frame #2 {
                    n369 = property on="Load parameters" class="Bool (strict)"("Val(Sgnl)"=TRUE ("Value (Signaling)")) -> ()  [unwired: 2 in, 2 out]
                  }
                  frame #3 {
                    n370 = Wait (ms)(milliseconds to wait=u32 200) -> ()  [unwired: 1 out]
                  }
                  frame #4 {
                    n371 = property on="Trap Raster Scan" class="Bool (strict)"("Val(Sgnl)"=TRUE ("Value (Signaling)")) -> ()  [unwired: 2 in, 2 out]
                  }
                  frame #5 {
                    n372 = Wait (ms)(milliseconds to wait=u32 2000) -> ()  [unwired: 1 out]
                  }
                  frame #6 {
                    n373 = while {
                      stop <- w641 stop-if-true
                      n374 = local read "Raster Scanning..."() -> (w643:bool)
                      n375 = local read "Saving..."() -> (w639:bool)
                      n376 = Wait (ms)(milliseconds to wait=u32 100) -> ()  [unwired: 1 out]
                      n377 = Not(x=w639) -> (.not. x?=w638:bool)
                      n378 = Not(x=w643) -> (.not. x?=w640:bool)
                      n379 = And(x=w640, y=w638) -> (x .and. y?=w641:bool)
                    }
                  }
                  frame #7 {
                    n380 = property on="Trap Delta (MHz)" class="DigNum (strict)"("Val(Sgnl)"=w644) -> ()  [unwired: 2 in, 2 out]
                  }
                }
              }
            }
          }
          frame #8 {
            n381 = local read "Save ave N"() -> (w646:dbl)
            n382 = case shown="False" "W/ Offset 2" {
              tunnel: w647 -> [_ w654]
              tunnel: w646 -> [_ w653]
              tunnel: w645 -> [w649 _]
              frame False {
                n383 = case shown="False" w649 {
                  frame False {
                    n384 = Multiply(x="Cal read wait (s)", y=u32 1000 ("milliseconds to wait")) -> (x*y=w651:u32)
                    n385 = Wait (ms)(milliseconds to wait=w651) -> ()  [unwired: 1 out]
                  }
                  frame True {
                  }
                }